vi "UHR-Fleezers Control (host) - 12.6.1.vi"() -> ()   [LabVIEW 2012] (continued)
                                n1136 = And(x=w1687, y=w1688) -> (x .and. y?=w1685:bool)
                                n1137 = And(x=w1686, y=w1688) -> (x .and. y?=w1684:bool)
                                n1138 = case shown="True" w1685 {
                                frame False {
                                }
                                frame True {
                                n1139 = local read "Confocal Y 2 (V)"() -> (w1694:dbl)
                                n1140 = local read "Confocal X 2 (V)"() -> (w1693:dbl)
                                n1141 = property on="AO2" class="Slide (strict)"("Val(Sgnl)"=w1693) -> ()  [unwired: 2 in, 2 out]
                                n1142 = property on="AO1" class="Slide (strict)"("Val(Sgnl)"=w1694) -> ()  [unwired: 2 in, 2 out]
                                }
                                }
                                n1143 = case shown="True" w1684 {
                                frame False {
                                }
                                frame True {
                                n1144 = local read "Confocal X 1 (V)"() -> (w1691:dbl)
                                n1145 = local read "Confocal Y 1 (V)"() -> (w1692:dbl)
                                n1146 = property on="AO1" class="Slide (strict)"("Val(Sgnl)"=w1692) -> ()  [unwired: 2 in, 2 out]
                                n1147 = property on="AO2" class="Slide (strict)"("Val(Sgnl)"=w1691) -> ()  [unwired: 2 in, 2 out]
                                }
                                }
                                }
                                frame #5 {
                                n1148 = Wait (ms)(milliseconds to wait=u32 1500) -> ()  [unwired: 1 out]
                                }
                                frame #6 {
                                n1149 = property on="Rem fb disp offset" class="Bool (strict)"("Val(Sgnl)"=TRUE ("Value (Signaling)")) -> ()  [unwired: 2 in, 2 out]
                                }
                                }
                                }
                                frame True {
                                n1150 = flat-sequence {
                                tunnel: w1697 -> [w1698]
                                frame #0 {
                                n1151 = property on="Trap Delta (MHz)" class="DigNum (strict)"("Val(Sgnl)"=w1698) -> ()  [unwired: 2 in, 2 out]
                                }
                                frame #1 {
                                n1152 = Wait (ms)(milliseconds to wait=u32 500) -> ()  [unwired: 1 out]
                                }
                                frame #2 {
                                n1153 = local read "Shift confocal"() -> (w1704:bool)
                                n1154 = local read "Mean"() -> (w1706:dbl)
                                n1155 = Greater?(x=w1706, y=11.0) -> (0:w1703:bool)
                                n1156 = Not(x=w1703) -> (.not. x?=w1702:bool)
                                n1157 = And(x=w1703, y=w1704) -> (x .and. y?=w1701:bool)
                                n1158 = And(x=w1702, y=w1704) -> (x .and. y?=w1700:bool)
                                n1159 = case shown="True" w1701 {
                                frame False {
                                }
                                frame True {
                                n1160 = local read "Confocal Y 2 (V)"() -> (w1710:dbl)
                                n1161 = local read "Confocal X 2 (V)"() -> (w1709:dbl)
                                n1162 = property on="AO2" class="Slide (strict)"("Val(Sgnl)"=w1709) -> ()  [unwired: 2 in, 2 out]
                                n1163 = property on="AO1" class="Slide (strict)"("Val(Sgnl)"=w1710) -> ()  [unwired: 2 in, 2 out]
                                }
                                }
                                n1164 = case shown="True" w1700 {
                                frame False {
                                }
                                frame True {
                                n1165 = local read "Confocal Y 1 (V)"() -> (w1708:dbl)
                                n1166 = local read "Confocal X 1 (V)"() -> (w1707:dbl)
                                n1167 = property on="AO2" class="Slide (strict)"("Val(Sgnl)"=w1707) -> ()  [unwired: 2 in, 2 out]
                                n1168 = property on="AO1" class="Slide (strict)"("Val(Sgnl)"=w1708) -> ()  [unwired: 2 in, 2 out]
                                }
                                }
                                }
                                }
                                }
                                }
                                }
                                }
                                }
                                }
                                n1169 = local read "Messages"() -> (w1656:string)
                                n1170 = Subtract(x=w1648, y=w1647) -> (x-y=w1654:dbl)
                                "Duration (s)" <- w1654
                                n1171 = Number To Decimal String(number=w1654, width (-)=i16 0) -> (decimal integer string=w1652:string)
                                n1172 = Concatenate Strings(w1652, " s fluorescence event." ("string")) -> (w1650:string)
                                n1173 = call "Update messages.vi"("Message to add"=w1650, "Old message string"=w1656) -> ("New message string"=w1655:string)
                                n1174 = local write "Reset Force"(FALSE ("Reset Force")) -> ()
                                n1175 = local write "Waiting"(TRUE ("Waiting")) -> ()
                                n1176 = local write "Messages"(w1655) -> ()
                                n1177 = local write "Fl. High"(FALSE ("Fl. High")) -> ()
                                n1178 = call <vilib>:"Beep.vi"() -> ()  [unwired: 3 in, 9 out]
                                }
                                }
                                n1179 = node-c288() -> ()  [unwired: 2 out]
                              }
                              n1180 = node-c288(w1624) -> ()  [unwired: 1 out]
                            }
                          }
                        }
                      }
                      n1181 = local read "Trap Delta (MHz)"() -> (w1539:dbl)
                      n1182 = local read "Trap Pos FB SP"() -> (w1534:fxp<+/-,16,1>)
                    }
                  }
                }
                frame #1 {
                  n1183 = local read "Stop All"() -> (w1720:bool)
                  n1184 = local read "Fl. Triggered..."() -> (w1718:bool)
                  n1185 = Not(x=w1718) -> (.not. x?=w1719:bool)
                  n1186 = Or(x=w1719, y=w1720) -> (x .or. y?=w1717:bool)
                }
              }
              n1187 = case shown="True" w1311 {
                frame False {
                }
                frame True {
                  n1188 = local read "Confocal Y 1 (V)"() -> (w1321:dbl)
                  n1189 = local read "Confocal X 1 (V)"() -> (w1320:dbl)
                  n1190 = property on="AO2" class="Slide (strict)"("Val(Sgnl)"=w1320) -> ()  [unwired: 2 in, 2 out]
                  n1191 = property on="AO1" class="Slide (strict)"("Val(Sgnl)"=w1321) -> ()  [unwired: 2 in, 2 out]
                }
              }
              n1192 = case shown="True" w1311 {
                frame False {
                }
                frame True {
                  w1319 = FALSE ("Fl. High")
                  n1193 = local write "Waiting"(w1319) -> ()
                  n1194 = local write "Fl. High"(w1319) -> ()
                }
              }
              n1195 = node-c288() -> ()  [unwired: 2 out]
            }
            n1196 = node-c288(w1309) -> ()  [unwired: 1 out]
          }
        }
      }
      event "Stop All": Value Change {
        n1197 = event-data() -> ()  [unwired: 7 out]
        n1198 = local read "Stop All"() -> (w1725:bool)
      }
    }
    n1199 = node-c288() -> ()  [unwired: 2 out]
  }
  n1200 = timed-loop "Basic control parameters (all FPGA settings, other basic controls)" {
    tunnel: w17 -> [w1734]
    shift-right: [w1733] -> _
    shift-left: errorcluster {"status"=FALSE, "code"=0, "source"=""} ("error out") -> [w1732]
    tunnel: [w1731] -> _
    timing: w127 -> [_]
    timing-out: [_] -> w126
    tunnel: w100 -> [w1730]
    tunnel: w72 -> [w1729]
    tunnel: w71 -> [w1728]
    tunnel: w70 -> [w1727]
    tunnel: w69 -> [w1726]
    stop <- w1731 stop-if-true
    n1201 = node-c288() -> ()  [unwired: 2 out]
    n1202 = event shown="[4] \"- phase (DIO)\", \"+ phase (AI1)\", \"- phase (AI1)\", \"Phase adj. (DIO)\", \"+ phase (DIO)\": Value Change" {
      selector: _ -> [_ _ _ _ _ _ _ _ _ _ _ _ _ _ _ _ _ _ _ _ _ _ _ _ _ _ _ _ _ _ _ _ _ _ _ _ _ _ _ _ _ _ _ _ _ _ _ _ _ _ _ _ _ _ _ _ _ _ _ _ _ _ _ _ _ _ _ _ _ _ _ _ _ _]
      dyn-events: _ -> [_ _ _ _ _ _ _ _ _ _ _ _ _ _ _ _ _ _ _ _ _ _ _ _ _ _ _ _ _ _ _ _ _ _ _ _ _ _ _ _ _ _ _ _ _ _ _ _ _ _ _ _ _ _ _ _ _ _ _ _ _ _ _ _ _ _ _ _ _ _ _ _ _ _]
      timeout: _ -> [_ _ _ _ _ _ _ _ _ _ _ _ _ _ _ _ _ _ _ _ _ _ _ _ _ _ _ _ _ _ _ _ _ _ _ _ _ _ _ _ _ _ _ _ _ _ _ _ _ _ _ _ _ _ _ _ _ _ _ _ _ _ _ _ _ _ _ _ _ _ _ _ _ _]
      tunnel: w1734 -> [w1775 _ _ _ w1819 _ w1841 _ _ _ _ w1907 _ _ w1950 w1956 w1963 w1968 w2041 _ w2057 w2082 w2103 w2124 w2144 w2173 w2199 w2202 w2206 w2301 w2306 w2344 _ w2379 w2383 w2394 w2398 w2402 _ w2410 _ _ _ _ _ _ _ _ _ _ _ _ _ _ _ _ _ w2788 _ w2805 _ w2812 w2830 _ w2837 w2845 w2860 w2876 w2882 _ w2891 _ w2910 _]
      tunnel: [w1774 _ _ _ w1809 _ w1840 _ _ w1872 _ w1886 _ _ w1949 w1952 w1962 w1965 w2035 _ w2056 w2081 w2101 w2122 w2142 w2167 w2197 _ w2204 w2299 w2304 w2342 _ w2377 w2381 w2385 w2396 w2400 _ w2408 _ _ _ _ _ _ _ _ _ _ _ _ _ _ _ _ _ w2786 _ _ _ _ w2827 _ _ _ _ _ _ _ _ _ _ _] -> w1733
      tunnel: w1732 -> [w1773 _ _ _ w1818 _ w1839 _ _ w1872 _ w1906 _ _ w1948 w1951 w1961 w1964 w2040 _ w2055 w2080 w2102 w2123 w2143 w2172 w2198 w2201 w2205 w2300 w2305 w2343 _ w2378 w2382 w2393 w2397 w2401 _ w2409 _ _ _ _ _ _ _ _ _ _ _ _ _ _ _ _ _ w2787 _ w2804 _ w2811 w2829 _ w2836 w2844 w2859 w2875 w2881 _ w2890 _ w2909 _]
      tunnel: [_ _ _ _ _ _ _ _ _ w1871 _ _ _ _ _ _ _ _ _ _ _ _ _ _ _ _ _ _ _ _ _ _ _ _ _ _ _ _ _ _ _ _ _ _ _ _ _ _ _ _ _ _ _ _ _ _ _ _ _ _ _ _ _ _ _ _ _ _ _ _ _ _ _ _] -> w1731
      tunnel: [_ _ _ _ _ _ _ "Round T1 X" _ _ _ _ _ _ _ _ _ _ _ _ _ _ _ _ _ _ _ _ _ _ _ _ _ _ _ _ _ _ _ _ _ _ _ _ _ _ _ _ _ _ _ _ _ _ _ _ _ _ _ _ _ _ _ _ _ _ _ _ _ _ _ _ _ _] -> _
      tunnel: [_ _ _ "Adjust Scale\nto Mean" _ _ _ _ _ _ _ _ _ _ _ _ _ _ _ _ _ _ _ _ _ _ _ _ "Test ttrig" _ _ _ _ _ _ _ _ _ _ _ _ _ _ _ _ _ _ "Flush Sample" "Flush Pump 3" "Flush Pump 1" "Clear Volume" _ _ _ _ _ _ _ _ _ _ _ _ _ _ _ _ _ _ _ _ _ _ _] -> _
      tunnel: [_ _ _ _ _ _ _ _ "Round T2 X" _ "Delayed Interlace Start" _ _ _ _ _ _ _ _ _ _ _ _ _ _ _ _ _ _ _ _ _ _ _ _ _ _ _ _ _ _ _ _ _ _ _ _ _ _ _ _ _ _ _ _ _ _ _ _ _ _ _ _ _ _ _ _ _ _ _ _ _ _ _] -> _
      tunnel: w1730 -> [_ _ _ _ _ _ _ _ _ _ _ _ _ _ _ _ _ _ _ _ _ _ _ _ _ _ _ _ _ _ _ _ _ _ _ _ _ _ _ _ _ _ _ w2567 w2574 w2581 w2586 w2595 _ _ w2701 _ _ _ _ _ _ _ _ _ _ _ _ _ _ _ _ _ _ _ _ _ _ _]
      tunnel: w1729 -> [_ _ _ _ _ _ _ _ _ _ _ _ _ _ _ _ _ _ _ _ _ _ _ _ _ _ _ _ _ _ _ _ _ _ _ _ _ _ _ _ _ w2484 _ _ _ _ _ _ w2639 _ _ w2707 _ w2716 _ w2730 _ _ _ _ _ _ _ _ _ _ _ _ _ _ _ _ _ _]
      tunnel: w1728 -> [_ _ _ _ _ _ _ _ _ _ _ _ _ _ _ _ _ _ _ _ _ _ _ _ _ _ _ _ _ _ _ _ _ _ _ _ _ _ _ _ _ _ _ _ _ _ _ _ _ _ _ _ _ _ _ _ _ _ _ _ _ _ _ _ _ _ _ _ _ _ _ _ _ _]
      tunnel: w1727 -> [_ _ _ _ _ _ _ _ _ _ _ _ _ _ _ _ _ _ _ _ _ _ _ _ _ _ _ _ _ _ _ _ _ _ _ _ _ _ _ _ w2421 _ _ _ _ _ _ _ _ w2669 _ _ w2712 _ w2723 _ w2755 _ _ _ _ _ _ _ _ _ _ _ _ _ _ _ _ _]
      tunnel: w1726 -> [_ _ _ _ _ _ _ _ _ _ _ _ _ _ _ _ _ _ _ _ _ _ _ _ _ _ _ _ _ _ _ _ _ _ _ _ _ _ _ _ _ _ _ _ _ _ _ _ _ _ _ _ _ _ _ _ _ _ _ _ _ _ _ _ _ _ _ _ _ _ _ _ _ _]
      event "AI Count (ticks)", "Sets to FIFO (Traps)", "Save ave N", "FPGA Ave.", "# Samples/channel", "N sets to save": Value Change {
        # "So that if 'Save ave N' is updated, the AOD scanning code updates too."
        n1203 = event-data() -> ()  [unwired: 6 out]
        n1204 = local read "AI Count (ticks)"() -> (w1757:u16)
        n1205 = Unbundle By Name("Sets to FIFO (Traps)") -> ("Set 1"=w1740:bool, "Set 2"=w1739:bool, "Set 3"=w1738:bool)
        n1206 = Boolean To (0,1)(Boolean="Sets to FIFO (Traps)") -> (0, 1=w1765:cluster{"Set 1":i16, "Set 2":i16, "Set 3":i16})
        n1207 = xnode "Read/Write Control"("FPGA VI Reference In"=w1775, "error in"=w1773, "ai count"=w1757, "Set 1"=w1740, "Set 2"=w1739, "Set 3"=w1738, "N of AI1 Int Acq Sets"="N Acq Sets (Traps + Fl.)") -> ("error out"=w1774:errorcluster)  [unwired: 1 out]
        n1208 = Cluster To Array(cluster=w1765) -> (array=w1764:i16[])
        n1209 = To Unsigned Long Integer(number=w1764) -> (unsigned 32bit integer=w1746:u32[])
        n1210 = local read "Scan steps (AOD)"() -> (w1766:u64)
        n1211 = Multiply(x=w1757, y="N Acq Sets (Traps + Fl.)") -> (x*y=w1755:u16)
        n1212 = Divide(x=40000000.0, y=w1757) -> (x/y=w1749:dbl)
        "AI rate (Hz)" <- w1749
        "Ave. Rate (Hz)" <- w1749
        n1213 = Add Array Elements(numeric array=w1746) -> (sum=w1758:u32)
        "Trap Sets" <- w1758
        n1214 = Reciprocal(x=w1749) -> (1/x=→"Ave. Period (s)":dbl)
        n1215 = property on="Scan steps (AOD)" class="DigNum (strict)"("Val(Sgnl)"=w1766) -> ()  [unwired: 2 in, 2 out]
        n1216 = Divide(x=w1749, y="N Acq Sets (Traps + Fl.)") -> (x/y=w1770:dbl)
        "Data Rate (Hz)" <- w1770
        n1217 = Reciprocal(x=w1770) -> (1/x=→"Data Period (s)":dbl)
        n1218 = local read "Save ave N"() -> (w1769:dbl)
        n1219 = Divide(x=w1770, y=w1769) -> (x/y=w1768:dbl)
        "Save Data Rate (Hz)" <- w1768
        n1220 = Reciprocal(x=w1768) -> (1/x=→"Save Data Period (s)":dbl)
        n1221 = Multiply(x=w1755, y="# Samples/trap") -> (x*y=w1753:u32)
        "Counts/DMA" <- w1753
        n1222 = property on="Trap Disp. Downsample" class="DigNum (strict)"("Maximum"="# Samples/trap") -> ()  [unwired: 2 in, 2 out]
        n1223 = Multiply(x=w1758, y="# Samples/trap") -> (x*y=w1747:u32)
        "# Samples/channel" <- w1747
        n1224 = Multiply(x=w1747, y=u32 8) -> (x*y=→"Trap AI Elements/DMA read":u32)
        n1225 = local read "APD Int. Count"() -> (w1754:u32)
        n1226 = Multiply(x=w1747, y=u32 3) -> (x*y=→"Trap Pos Elements/DMA read":u32)
        n1227 = Divide(x=w1753, y=w1754) -> (x/y=w1744:dbl)
        "APD Samples/FIFO Acq." <- w1744
        n1228 = Divide(x=w1753, y=40000000.0) -> (x/y=w1751:dbl)
        "DMA Update Period (s)" <- w1751
        n1229 = local read "Number of APDs"() -> (w1737:u8)
        n1230 = Multiply(x=w1737, y=w1744) -> (x*y=→"APD Elements/DMA read":dbl)
        n1231 = property on="APD Disp. Downsample" class="DigNum (strict)"("Maximum"=w1744) -> ()  [unwired: 2 in, 2 out]
        n1232 = local read "N sets to save"() -> (w1763:u32)
        n1233 = Multiply(x=w1751, y=w1763) -> (x*y=→"Total Time (s)":dbl)
        "FPGA Averaging" <- FALSE ("FPGA Averaging")
      }
      event "Remove Offset": Value Change {
        n1234 = event-data() -> ()  [unwired: 7 out]
        n1235 = local write "Remove Offset"(FALSE ("Remove Offset")) -> ()
        n1236 = local read "Bead Mean (nm)"() -> (w1777:dbl)
        n1237 = local read "Offset (nm)"() -> (w1778:dbl)
        n1238 = Add(x=w1777, y=w1778) -> (x+y=w1776:dbl)
        n1239 = local write "Offset (nm)"(w1776) -> ()
        n1240 = disable-structure shown="Disabled" {
          frame Disabled {
            n1241 = local read "Bead Mean (nm)"() -> (w1783:dbl)
            n1242 = Add(y=w1783) -> (x=w1782:dbl, x+y=w1781:dbl)
            n1243 = Subtract(x=w1783, y=w1782) -> (x-y=w1780:dbl)
            n1244 = property on="Bead Separation" class="WFChart (strict)"("YScale.Minimum"=w1780) -> ()  [unwired: 2 in, 2 out]
            n1245 = property on="Bead Separation" class="WFChart (strict)"("YScale.Maximum"=w1781) -> ()  [unwired: 2 in, 2 out]
          }
          frame Enabled {
          }
        }
      }
      event "Detector Type": Value Change {
        n1246 = event-data() -> ()  [unwired: 7 out]
        n1247 = local read "AI labels"() -> (w1784:string[])
        n1248 = property on="High Res. Display" class="Ring (strict)"("Strings []"=w1784) -> ()  [unwired: 2 in, 2 out]
        n1249 = Build Array (concatenate)(w1784, "none") -> (w1785:string[])
        n1250 = property on="FFT 1 Choice 1" class="Ring (strict)"("Strings []"=w1785) -> ()  [unwired: 2 in, 2 out]
        n1251 = property on="FFT 1 Choice 2" class="Ring (strict)"("Strings []"=w1785) -> ()  [unwired: 2 in, 2 out]
        n1252 = property on="FFT 2 Choice 1" class="Ring (strict)"("Strings []"=w1785) -> ()  [unwired: 2 in, 2 out]
        n1253 = property on="FFT 2 Choice 2" class="Ring (strict)"("Strings []"=w1785) -> ()  [unwired: 2 in, 2 out]
        n1254 = Bundle("APD 1", "APD 2") -> (w1788:cluster{string, string})  [unwired: 1 out]
        n1255 = Cluster To Array(cluster=w1788) -> (array=w1786:string[])
        n1256 = Build Array (concatenate)(w1786, w1785) -> (w1790:string[])
        n1257 = Array Size(array=w1790) -> (size(s)=w1791:i32)
        n1258 = property on="Signals to Plot" class="LstBox (strict)"("Item Names"=w1790) -> ()  [unwired: 2 in, 2 out]
        n1259 = property on="Signals to Plot" class="LstBox (strict)"("Number of Rows"=w1791) -> ()  [unwired: 2 in, 2 out]
        n1260 = property on="All Signals" class="WFChart (strict)"("LegNumRows"=w1791) -> ()  [unwired: 2 in, 2 out]
      }
      event "Adjust Scale\nto Mean": Value Change {
        n1261 = event-data() -> ()  [unwired: 7 out]
        n1262 = local read "APD 1 Rate (Hz)"() -> (w1800:dbl)
        n1263 = Multiply(x=1000.0, y="Above (kHz)") -> (x*y=w1798:dbl)
        n1264 = Multiply(x=1000.0, y="Below (kHz)") -> (x*y=w1796:dbl)
        n1265 = Add(x=w1798, y=w1800) -> (x+y=w1793:dbl)
        n1266 = Subtract(x=w1800, y=w1796) -> (x-y=w1794:dbl)
        n1267 = property on="APD Chart" class="WFChart (strict)"("YScale.Minimum"=w1794) -> ()  [unwired: 2 in, 2 out]
        n1268 = property on="APD Chart" class="WFChart (strict)"("YScale.Maximum"=w1793) -> ()  [unwired: 2 in, 2 out]
      }
      event "- phase (DIO)", "+ phase (AI1)", "- phase (AI1)", "Phase adj. (DIO)", "+ phase (DIO)": Value Change {
        # "digital phase (controls switching phase of AOM/AOD)"
        # "Analog phase"
        n1269 = event-data() -> ()  [unwired: 7 out]
        n1270 = Negate(x="Phase adj. (AI1)") -> (-x=w1816:i16)
        n1271 = Negate(x="Phase adj. (DIO)") -> (-x=w1805:i16)
        n1272 = Select(t=w1816, s="- phase (AI1)", f="Phase adj. (AI1)") -> (s? t:f=w1815:i16)
        n1273 = Select(t=w1805, s="- phase (DIO)", f="Phase adj. (DIO)") -> (s? t:f=w1804:i16)
        n1274 = xnode "Read/Write Control"("FPGA VI Reference In"=w1819, "error in"=w1818, "Phase count adjustment"=w1815, "Phase count adjustment (DIO)"=w1804) -> ("FPGA VI Reference Out"=w1814:T20, "error out"=w1813:errorcluster)
        n1275 = Or(x="- phase (AI1)", y="+ phase (AI1)") -> (x .or. y?=w1810:bool)
        n1276 = Or(x="- phase (DIO)", y="+ phase (DIO)") -> (x .or. y?=w1808:bool)
        n1277 = xnode "Read/Write Control"("FPGA VI Reference In"=w1814, "error in"=w1813, "+ phase"=w1810, "+ phase (DIO)"=w1808) -> ("error out"=w1809:errorcluster)  [unwired: 1 out]
      }
      event "Signals to Plot": Double Click {
        w1822 = u32 9868950 ("Color Box")
        n1278 = event-data() -> ("Row"=w1824:i32)  [unwired: 9 out]
        n1279 = property on="All Signals" class="WFChart (strict)"("Active Plot"=w1824) -> (error out=w1835:errorcluster)  [unwired: 2 in, 1 out]
        n1280 = property on="All Signals" class="WFChart (strict)" props=["Plot", "Visible?", "Plot", "Plot Color"](error in=w1835) -> (error out=w1834:errorcluster, "Plot.Visible?"=w1833:bool)  [unwired: 1 in, 2 out]
        n1281 = Select(t=FALSE ("Plot.Visible"), s=w1833, f=TRUE ("Plot.Visible")) -> (s? t:f=w1828:bool)
        n1282 = property on="All Signals" class="WFChart (strict)"(error in=w1834, "Plot.Visible?"=w1828) -> (error out=w1830:errorcluster)  [unwired: 1 in, 1 out]
        n1283 = property on="All Signals" class="WFChart (strict)"(error in=w1830) -> (error out=w1825:errorcluster, "Plot.Plot Color"=w1829:u32)  [unwired: 1 in, 1 out]
        n1284 = property on="Signals to Plot" class="LstBox (strict)"(error in=w1825, "Active Row"=w1824) -> (error out=w1823:errorcluster)  [unwired: 1 in, 1 out]
        n1285 = Select(t=w1829, s=w1828, f=u32 0) -> (s? t:f=w1826:u32)
        n1286 = property on="Signals to Plot" class="LstBox (strict)"(error in=w1823, "CellFontColor"=w1826, "SelColor"=w1822, "CellBG"=w1822, "CellFontSize"=u32 20 ("Active Row:Cell Font:Size"), "CellFontBold"=TRUE ("Active Row:Cell Font:Bold")) -> ()  [unwired: 1 in, 2 out]
      }
      event "BD 1 Frequency 1 (MHz)", "BD 1 Frequency 2 (MHz)", "BD 1 Frequency 3 (MHz)", "BD 2 Frequency 1 (MHz)", "BD 2 Frequency 2 (MHz)", "BD 2 Frequency 3 (MHz)", "Trap Delta (MHz)": Value Change {
        n1287 = event-data() -> ("CtlRef"=w1838:refnum<vi>)  [unwired: 6 out]
        n1288 = control-ref of="Trap Delta (MHz)"() -> (w1837:refnum<vi>)
        n1289 = Equal?(x=w1837, y=w1838) -> (x = y?=w1836:bool)
        n1290 = case shown="False" "Oscillate Set 1" {
          tunnel: w1841 -> [w1861 _]
          tunnel: [w1860 w1864] -> w1840
          tunnel: w1839 -> [w1859 w1864]
          tunnel: w1836 -> [w1844 _]
          frame False {
            n1291 = local read "BD 1 Frequency 2 (MHz)"() -> (w1848:dbl)
            n1292 = local read "BD 1 Frequency 1 (MHz)"() -> (w1846:dbl)
            n1293 = Subtract(x=w1848, y="Trap Delta (MHz)") -> (x-y=w1845:dbl)
            n1294 = Select(t=w1845, s=w1844, f=w1846) -> (s? t:f=w1843:dbl)
            n1295 = local read "Y RF Frequency Limits (MHz)"() -> (w1849:T16)
            n1296 = local read "X RF Frequency Limits (MHz)"() -> (w1850:T16)
            n1297 = local read "BD 1 Frequency 3 (MHz)"() -> (w1862:dbl)
            n1298 = local write "BD 1 Frequency 1 (MHz)"(w1843) -> ()
            n1299 = local read "BD 2 Frequency 1 (MHz)"() -> (w1853:dbl)
            n1300 = local read "BD 2 Frequency 2 (MHz)"() -> (w1852:dbl)
            n1301 = local read "BD 2 Frequency 3 (MHz)"() -> (w1863:dbl)
            n1302 = call "set RF board frequency - interlace.vi"("Board 2 Frequency Limits"=w1849, "Board 1 Frequency Limits"=w1850, "error in"=w1859, "FPGA VI Reference In"=w1861, "Board 2 Frequency 3 (MHz)"=w1863, "Board 1 Frequency 3 (MHz)"=w1862, "Board 2 Frequency 2 (MHz)"=w1852, "Board 2 Frequency 1 (MHz)"=w1853, "Board 1 Frequency 2 (MHz)"=w1848, "Board 1 Frequency 1  (MHz)"=w1843) -> ("error out"=w1860:errorcluster)  [unwired: 1 out]
            n1303 = Subtract(x=w1853, y=w1852) -> (x-y=w1857:dbl)
            n1304 = Subtract(x=w1843, y=w1848) -> (x-y=w1858:dbl)
            n1305 = Square(x=w1857) -> (x^2=w1855:dbl)
            n1306 = Square(x=w1858) -> (x^2=w1856:dbl)
            n1307 = Add(x=w1856, y=w1855) -> (x+y=w1854:dbl)
            n1308 = Square Root(x=w1854) -> (sqrt(x)=w1851:dbl)
            n1309 = local write "Trap Delta (MHz)"(w1851) -> ()
            n1310 = property on="Initial delta (MHz)" class="DigNum (strict)"("Val(Sgnl)"=w1851) -> ()  [unwired: 2 in, 2 out]
          }
          frame True {
          }
        }
      }
      event "Round T1 X": Value Change {
        n1311 = event-data() -> ()  [unwired: 7 out]
        n1312 = local read "BD 1 Frequency 1 (MHz)"() -> (w1867:dbl)
        n1313 = Round To Nearest(number=w1867) -> (nearest integer value=w1866:dbl)
        n1314 = property on="BD 1 Frequency 1 (MHz)" class="DigNum (strict)"("Val(Sgnl)"=w1866) -> ()  [unwired: 2 in, 2 out]
      }
      event "Round T2 X": Value Change {
        n1315 = event-data() -> ()  [unwired: 7 out]
        n1316 = local read "BD 1 Frequency 2 (MHz)"() -> (w1869:dbl)
        n1317 = Round To Nearest(number=w1869) -> (nearest integer value=w1868:dbl)
        n1318 = property on="BD 1 Frequency 2 (MHz)" class="DigNum (strict)"("Val(Sgnl)"=w1868) -> ()  [unwired: 2 in, 2 out]
      }
      event "Stop All": Value Change {
        n1319 = event-data() -> ()  [unwired: 7 out]
        n1320 = local read "Stop All"() -> (w1871:bool)
      }
      event "Delayed Interlace Start": Value Change {
        n1321 = event-data() -> ()  [unwired: 7 out]
        n1322 = flat-sequence {
          frame #0 {
            n1323 = Multiply(x="Delay to Interlace (s)", y=1000.0) -> (x*y=w1874:dbl)
            n1324 = Wait (ms)(milliseconds to wait=w1874) -> ()  [unwired: 1 out]
          }
          frame #1 {
            n1325 = property on="Laser interlacing mode" class="RadioBtnsControl (strict)"("Val(Sgnl)"=enum32{"Laser ON", "Laser OFF", "Interlace"}."Interlace" ("Value (Signaling)")) -> ()  [unwired: 2 in, 2 out]
          }
        }
      }
      event "BD 1 Amplitude 1 (%)", "BD 1 Amplitude 2 (%)", "BD 1 Amplitude 3 (%)", "BD 2 Amplitude 1 (%)", "BD 2 Amplitude 2 (%)", "BD 2 Amplitude 3 (%)", "Trap 1 ON", "Trap 2 ON", "Trap 3 ON", "Feedback On/Off", "All FB On/Off": Value Change {
        w1898 = i16 1 ("f")
        n1326 = event-data() -> ()  [unwired: 7 out]
        n1327 = local write "Trap 1 (ON/OFF)"("Trap 1 ON") -> ()
        n1328 = local write "Trap 2 (ON/OFF)"("Trap 2 ON") -> ()
        n1329 = Boolean To (0,1)(Boolean="Trap 3 ON") -> (0, 1=w1899:i16)
        n1330 = Boolean To (0,1)(Boolean="Trap 1 ON") -> (0, 1=w1900:i16)
        n1331 = Boolean To (0,1)(Boolean="Trap 2 ON") -> (0, 1=w1901:i16)
        n1332 = Select(t=w1901, s="Trap ON/OFF X or Y Amp?", f=w1898) -> (s? t:f=w1896:i16)
        n1333 = Select(t=w1900, s="Trap ON/OFF X or Y Amp?", f=w1898) -> (s? t:f=w1897:i16)
        n1334 = Select(t=w1899, s="Trap ON/OFF X or Y Amp?", f=w1898) -> (s? t:f=w1895:i16)
        n1335 = Select(t=w1898, s="Trap ON/OFF X or Y Amp?", f=w1901) -> (s? t:f=w1893:i16)
        n1336 = Select(t=w1898, s="Trap ON/OFF X or Y Amp?", f=w1900) -> (s? t:f=w1894:i16)
        n1337 = Select(t=w1898, s="Trap ON/OFF X or Y Amp?", f=w1899) -> (s? t:f=w1892:i16)
        n1338 = And(x="All FB On/Off", y="Feedback On/Off") -> (x .and. y?=w1890:cluster{"Set 1":bool, "Set 2":bool})
        n1339 = local read "BD 1 Amplitude 1 (%)"() -> (w1910:dbl)
        n1340 = local read "BD 1 Amplitude 2 (%)"() -> (w1909:dbl)
        n1341 = local read "BD 1 Amplitude 3 (%)"() -> (w1908:dbl)
        n1342 = Unbundle By Name(w1890) -> ("Set 1"=w1885:bool, "Set 2"=w1882:bool)
        n1343 = local read "Y RF Amplitude Limits (%)"() -> (w1878:T16)
        n1344 = local read "X RF Amplitude Limits (%)"() -> (w1879:T16)
        n1345 = local read "BD 2 Amplitude 1 (%)"() -> (w1911:dbl)
        n1346 = local read "BD 2 Amplitude 2 (%)"() -> (w1912:dbl)
        n1347 = local read "BD 2 Amplitude 3 (%)"() -> (w1913:dbl)
        n1348 = And(x="Trap 2 ON", y=w1882) -> (x .and. y?=w1880:bool)
        n1349 = And(x="Trap 1 ON", y=w1885) -> (x .and. y?=w1883:bool)
        n1350 = Multiply(x=w1897, y=w1910) -> (x*y=w1905:dbl)
        n1351 = Multiply(x=w1909, y=w1896) -> (x*y=w1903:dbl)
        n1352 = Multiply(x=w1908, y=w1895) -> (x*y=w1904:dbl)
        n1353 = Multiply(x=w1911, y=w1894) -> (x*y=w1914:dbl)
        n1354 = Multiply(x=w1912, y=w1893) -> (x*y=w1915:dbl)
        n1355 = Multiply(x=w1913, y=w1892) -> (x*y=w1916:dbl)
        n1356 = call "set RF board amplitude - interlace.vi"("Board 2 Amplitude Limits"=w1878, "Board 1 Amplitude Limits"=w1879, "error in"=w1906, "FPGA VI Reference In"=w1907, "Board 2 Amplitude 3 (%)"=w1916, "Board 1 Amplitude 3 (%)"=w1904, "Board 2 Amplitude 2 (%)"=w1915, "Board 2 Amplitude 1 (%)"=w1914, "Board 1 Amplitude 2 (%)"=w1903, "Board 1 Amplitude 1 (%)"=w1905) -> ("error out"=w1887:errorcluster, "FPGA VI Reference Out"=w1888:T20)
        n1357 = xnode "Read/Write Control"("FPGA VI Reference In"=w1888, "error in"=w1887, "FB On/Off Set 1"=w1883, "FB On/Off Set 2"=w1880) -> ("error out"=w1886:errorcluster)  [unwired: 1 out]
      }
      event "Load parameters": Value Change {
        n1358 = event-data() -> ()  [unwired: 7 out]
        n1359 = property on="Saved AOD Raster Scan Parameter Sets" class="Arr (strict)"() -> ("Index Values"=w1927:u32[])  [unwired: 2 in, 2 out]
        n1360 = Index Array(array=w1927, index=0) -> (element=w1924:u32)
        n1361 = local write "Load parameters"(FALSE ("Load parameters")) -> ()
        n1362 = Index Array(array="Saved AOD Raster Scan Parameter Sets", index=w1924) -> (element=w1923:T30)
        n1363 = Unbundle By Name(w1923) -> ("Scan Range AOD (nm) 2"=w1922:dbl, "Step Size AOD (nm) 2"=w1921:dbl, "Scan Speed AOD (nm/s) 2"=w1920:dbl, "Number of scans (AOD) 2"=w1919:u16)
        n1364 = flat-sequence {
          tunnel: w1922 -> [w1930]
          tunnel: w1921 -> [w1929]
          tunnel: w1920 -> [w1928]
          tunnel: w1919 -> [w1931]
          frame #0 {
            n1365 = local write "Scan Speed (nm/s)"(w1928) -> ()
            n1366 = local write "Scan Range (nm)"(w1930) -> ()
            n1367 = local write "Step Size (nm)"(w1929) -> ()
          }
          frame #1 {
            n1368 = property on="Number of F/B Scans (AOD)" class="DigNum (strict)"("Val(Sgnl)"=w1931) -> ()  [unwired: 2 in, 2 out]
          }
        }
      }
      event "Trap 1 (ON/OFF)", "Trap 2 (ON/OFF)": Value Change {
        n1369 = event-data() -> ()  [unwired: 7 out]
        n1370 = property on="Trap 2 ON" class="Bool (strict)"("Val(Sgnl)"="Trap 2 (ON/OFF)") -> ()  [unwired: 2 in, 2 out]
        n1371 = property on="Trap 1 ON" class="Bool (strict)"("Val(Sgnl)"="Trap 1 (ON/OFF)") -> ()  [unwired: 2 in, 2 out]
      }
      event "DIO count 1 (ticks)", "DIO count 2 (ticks)", "DIO count 3 (ticks)", "Interlace", "Number Interlace Sets", "Not-Interlacing Set": Value Change {
        n1372 = event-data() -> ()  [unwired: 7 out]
        n1373 = local read "DIO count 3 (ticks)"() -> (w1944:u16)
        n1374 = local read "DIO count 1 (ticks)"() -> (w1946:u16)
        n1375 = local read "DIO count 2 (ticks)"() -> (w1945:u16)
        n1376 = To Unsigned Byte Integer(number="Not-Interlacing Set") -> (unsigned 8bit integer=w1935:u8)
        n1377 = Add(x=w1935, y=u8 1) -> (x+y=w1939:u8)
        n1378 = xnode "Read/Write Control"("FPGA VI Reference In"=w1950, "error in"=w1948, "DIO count 1 (ticks)"=w1946, "DIO count 2 (ticks)"=w1945, "DIO count 3 (ticks)"=w1944, "Interlace ON/OFF"="Interlace", "Number Interlace Cycles"="Number Interlace Sets", "Interlace Off Parameters"=w1939) -> ("error out"=w1949:errorcluster)  [unwired: 1 out]
        n1379 = Build Array(w1946, w1945, w1944) -> (w1937:u16[])
        n1380 = Split 1D Array(array=w1937, index="Number Interlace Sets") -> (first subarray=w1947:u16[])  [unwired: 1 out]
        n1381 = Index Array(array=w1937, index=w1935) -> (element=w1936:u16)
        n1382 = Add Array Elements(numeric array=w1947) -> (sum=w1941:u16)
        n1383 = Select(t=w1941, s="Interlace", f=w1936) -> (s? t:f=→"Total Counts (ticks)":u16)
      }
      event "Reset Feedback": Value Change {
        n1384 = event-data() -> ()  [unwired: 7 out]
        n1385 = Unbundle By Name("Reset Feedback") -> ("Set 1"=w1954:bool, "Set 2"=w1953:bool)
        n1386 = xnode "Read/Write Control"("FPGA VI Reference In"=w1956, "error in"=w1951, "FB Reset Set 1"=w1954, "FB Reset Set 2"=w1953) -> ("error out"=w1952:errorcluster)  [unwired: 1 out]
      }
      event "Trap Intensity PID Gains": Value Change {
        n1387 = event-data() -> ()  [unwired: 7 out]
        n1388 = Unbundle By Name("Trap Intensity PID Gains") -> ("proportional gain (Kc)"=w1959:i16, "integral gain (Kc*Ts/Ti)"=w1958:i16, "derivative gain (Kc*Td/Ts)"=w1957:i16)
        n1389 = xnode "Read/Write Control"("FPGA VI Reference In"=w1963, "error in"=w1961, "P1"=w1959, "I1"=w1958, "D1"=w1957) -> ("error out"=w1962:errorcluster)  [unwired: 1 out]
      }
      event "AI2 to Setpoint", "Setpoints (V)": Value Change {
        n1390 = event-data() -> ()  [unwired: 7 out]
        n1391 = xnode "Read/Write Control"("FPGA VI Reference In"=w1968, "error in"=w1964) -> ("FPGA VI Reference Out"=w1967:T20, "error out"=w1966:errorcluster, "AI2 Y Sum Set 1"=w1975:i16, "AI2 Y Sum Set 2"=w1974:i16)
        n1392 = Cluster To Array(cluster="AI2 to Setpoint") -> (array=w1978:bool[])
        n1393 = local read "AI2 (V)"() -> (w1976:cluster{"Set 1":dbl, "Set 2":dbl})
        n1394 = Or Array Elements(Boolean array=w1978) -> (logical OR=w1979:bool)
        n1395 = Bundle By Name(cluster=w1976, "Set 1"=w1975, "Set 2"=w1974) -> (w1973:cluster{"Set 1":dbl, "Set 2":dbl})
        n1396 = Divide(x=w1973, y=3276.7) -> (x/y=w1972:cluster{"Set 1":dbl, "Set 2":dbl})
        "AI2 (V)" <- w1972
        n1397 = case shown="True" w1979 {
          tunnel: [w1982 w1999] -> w1971
          tunnel: "AI2 to Setpoint" -> [_ w1995]
          tunnel: "Setpoints (V)" -> [w1983 w1998]
          tunnel: w1972 -> [_ w1992]
          frame False {
            n1398 = Multiply(x=3276.7, y=w1983) -> (x*y=w1984:cluster{"Set 1":dbl, "Set 2":dbl})
            n1399 = To Word Integer(number=w1984) -> (16bit integer=w1982:cluster{"Set 1":i16, "Set 2":i16})
          }
          frame True {
            n1400 = Unbundle By Name(w1992) -> ("Set 1"=w1991:dbl, "Set 2"=w1990:dbl)
            n1401 = Unbundle By Name(w1998) -> ("Set 1"=w1997:dbl, "Set 2"=w1996:dbl)
            n1402 = Unbundle By Name(w1995) -> ("Set 1"=w1994:bool, "Set 2"=w1993:bool)
            n1403 = Select(t=w1991, s=w1994, f=w1997) -> (s? t:f=w1989:dbl)
            n1404 = Select(t=w1990, s=w1993, f=w1996) -> (s? t:f=w1988:dbl)
            n1405 = Bundle By Name(cluster=w1998, "Set 1"=w1989, "Set 2"=w1988) -> (w1986:cluster{"Set 1":dbl, "Set 2":dbl})
            n1406 = local write "Setpoints (V)"(w1986) -> ()
            n1407 = Multiply(x=3276.7, y=w1986) -> (x*y=w1987:cluster{"Set 1":dbl, "Set 2":dbl})
            n1408 = To Word Integer(number=w1987) -> (16bit integer=w1999:cluster{"Set 1":i16, "Set 2":i16})
          }
        }
        n1409 = Unbundle By Name(w1971) -> ("Set 1"=w1970:i16, "Set 2"=w1969:i16)
        n1410 = xnode "Read/Write Control"("FPGA VI Reference In"=w1967, "error in"=w1966, "FB Setpoint Set 1"=w1970, "FB Setpoint Set 2"=w1969) -> ("error out"=w1965:errorcluster)  [unwired: 1 out]
      }
      event "+ phase (GI)", "- phase (GI)", "+ phase (GI) 2", "- phase (GI) 2", "+ phase (RI)", "- phase (RI)", "+ phase (Green FB)", "- phase (Green FB)": Value Change {
        n1411 = event-data() -> ()  [unwired: 7 out]
        n1412 = Or(x="+ phase (GI)", y="- phase (GI)") -> (x .or. y?=w2034:bool)
        n1413 = Negate(x="Phase adj. (GI)") -> (-x=w2039:i16)
        n1414 = Select(t=w2039, s="+ phase (GI)", f="Phase adj. (GI)") -> (s? t:f=w2038:i16)
        n1415 = Or(x="+ phase (GI) 2", y="- phase (GI) 2") -> (x .or. y?=w2025:bool)
        n1416 = Negate(x="Phase adj. (GI) 2") -> (-x=w2030:i16)
        n1417 = Select(t=w2030, s="+ phase (GI) 2", f="Phase adj. (GI) 2") -> (s? t:f=w2026:i16)
        n1418 = Negate(x="Phase adj. (RI)") -> (-x=w2024:i16)
        n1419 = Or(x="+ phase (RI)", y="- phase (RI)") -> (x .or. y?=w2020:bool)
        n1420 = Select(t=w2024, s="+ phase (RI)", f="Phase adj. (RI)") -> (s? t:f=w2019:i16)
        n1421 = Or(x="+ phase (Green FB)", y="- phase (Green FB)") -> (x .or. y?=w2013:bool)
        n1422 = Negate(x="Phase adj. (Green FB)") -> (-x=w2018:i16)
        n1423 = Select(t=w2018, s="+ phase (Green FB)", f="Phase adj. (Green FB)") -> (s? t:f=w2014:i16)
        n1424 = Negate(x="Phase adj. (BI AO)") -> (-x=w2012:i16)
        n1425 = Or(x="+ phase (BI AO)", y="- phase (BI AO)") -> (x .or. y?=w2002:bool)
        n1426 = Select(t=w2012, s="+ phase (BI AO)", f="Phase adj. (BI AO)") -> (s? t:f=w2004:i16)
        n1427 = Negate(x="Phase adj. (BI DO)") -> (-x=w2008:i16)
        n1428 = Or(x="+ phase (BI DO)", y="- phase (BI DO)") -> (x .or. y?=w2001:bool)
        n1429 = Select(t=w2008, s="+ phase (BI DO)", f="Phase adj. (BI DO)") -> (s? t:f=w2003:i16)
        n1430 = xnode "Read/Write Control"("FPGA VI Reference In"=w2041, "error in"=w2040, "Phase count adjustment (GI)"=w2038, "Phase count adjustment (GI) 2"=w2026, "Phase count adjustment (RI)"=w2019, "Phase count adjustment (Green FB)"=w2014, "Phase count adjustment (BI AO)"=w2004, "Phase count adjustment (BI D)"=w2003) -> ("FPGA VI Reference Out"=w2036:T20, "error out"=w2037:errorcluster)
        n1431 = xnode "Read/Write Control"("FPGA VI Reference In"=w2036, "error in"=w2037, "+ phase (GI)"=w2034, "+ phase (GI) 2"=w2025, "+ phase (RI)"=w2020, "+ phase (Green FB)"=w2013, "+ phase (BI AO)"=w2002, "+ phase (BI D)"=w2001) -> ("error out"=w2035:errorcluster)  [unwired: 1 out]
      }
      event "Green Laser ON/OFF", "Red Laser ON/OFF", "Blue Laser ON/OFF": Value Change {
        # "This loop shouldn't be initialized.  The main 'laser ON' settings should dominate and set the others."
        n1432 = event-data() -> ()  [unwired: 7 out]
        n1433 = property on="Red Laser ON" class="Bool (strict)"("Val(Sgnl)"="Red Laser ON/OFF") -> ()  [unwired: 2 in, 2 out]
        n1434 = property on="Blue Laser ON" class="Bool (strict)"("Val(Sgnl)"="Blue Laser ON/OFF") -> ()  [unwired: 2 in, 2 out]
        n1435 = property on="Green Laser ON" class="Bool (strict)"("Val(Sgnl)"="Green Laser ON/OFF") -> ()  [unwired: 2 in, 2 out]
      }
      event "Laser interlacing mode", "Green Laser ON", "Red Laser ON", "Blue Laser ON": Value Change {
        n1436 = event-data() -> ()  [unwired: 7 out]
        n1437 = local write "Green Laser ON/OFF"("Green Laser ON") -> ()
        n1438 = local write "Blue Laser ON/OFF"("Blue Laser ON") -> ()
        n1439 = local write "Red Laser ON/OFF"("Red Laser ON") -> ()
        n1440 = case shown="True" "Green Laser ON" {
          tunnel: "Laser interlacing mode" -> [_ w2078]
          tunnel: [enum32{"Laser ON", "Laser OFF", "Interlace"}."Laser OFF" ("Green laser mode") w2078] -> w2054
          tunnel: [FALSE w2074] -> w2053
          frame False {
          }
          frame True {
            n1441 = local read "Green FB On/Off"() -> (w2075:bool)
            n1442 = Equal?(x=w2078, y=enum32{"Laser ON", "Laser OFF", "Interlace"}."Interlace") -> (x = y?=w2076:bool)
            n1443 = And(x=w2076, y=w2075) -> (x .and. y?=w2074:bool)
          }
        }
        n1444 = case shown="True" "Red Laser ON" {
          tunnel: "Laser interlacing mode" -> [_ w2071]
          tunnel: [enum32{"Laser ON", "Laser OFF", "Interlace"}."Laser OFF" ("Green laser mode") w2071] -> w2050
          tunnel: [FALSE w2067] -> w2049
          frame False {
          }
          frame True {
            n1445 = local read "Red FB On/Off"() -> (w2068:bool)
            n1446 = Equal?(x=w2071, y=enum32{"Laser ON", "Laser OFF", "Interlace"}."Interlace") -> (x = y?=w2069:bool)
            n1447 = And(x=w2069, y=w2068) -> (x .and. y?=w2067:bool)
          }
        }
        n1448 = case shown="True" "Blue Laser ON" {
          tunnel: "Laser interlacing mode" -> [_ w2062]
          tunnel: [enum32{"Laser ON", "Laser OFF", "Interlace"}."Laser OFF" ("Green laser mode") w2062] -> w2046
          tunnel: [FALSE w2060] -> w2045
          frame False {
          }
          frame True {
            n1449 = local read "Blue FB On/Off"() -> (w2061:bool)
            n1450 = Equal?(x=w2062, y=enum32{"Laser ON", "Laser OFF", "Interlace"}."Interlace") -> (x = y?=w2063:bool)
            n1451 = And(x=w2063, y=w2061) -> (x .and. y?=w2060:bool)
          }
        }
        n1452 = xnode "Read/Write Control"("FPGA VI Reference In"=w2057, "error in"=w2055, "Operating Mode"=w2054, "Operating Mode 2"=w2054, "Green FB On/Off"=w2053, "Red Laser Operating Mode"=w2050, "RI Operating Mode 2"=w2050, "Red FB On/Off"=w2049, "BI Operating Mode (AO)"=w2046, "Blue Laser Operating Mode (D)"=w2046, "Blue FB On/Off"=w2045) -> ("error out"=w2056:errorcluster)  [unwired: 1 out]
      }
      event "Invert laser interlacing": Value Change {
        n1453 = event-data() -> ()  [unwired: 7 out]
        n1454 = xnode "Read/Write Control"("FPGA VI Reference In"=w2082, "error in"=w2080, "Invert GI"="Invert laser interlacing", "Invert GI 2"="Invert laser interlacing", "Invert RI"="Invert laser interlacing", "Invert RI 2"="Invert laser interlacing", "Invert BI (AO)"="Invert laser interlacing", "Invert BI (D)"="Invert laser interlacing") -> ("error out"=w2081:errorcluster)  [unwired: 1 out]
      }
      event "Green FB Setpoint (mV)", "Green FB Gains", "Green FB On/Off", "Green Intensity % (FB OFF)", "Green int current ON count adj": Value Change {
        n1455 = event-data() -> ()  [unwired: 7 out]
        n1456 = local read "Green FB Setpoint (mV)"() -> (w2093:dbl)
        n1457 = Multiply(x=w2093, y=3.2767) -> (x*y=w2092:dbl)
        n1458 = local read "Green Intensity % (FB OFF)"() -> (w2096:dbl)
        n1459 = Multiply(x=w2096, y=655.35) -> (x*y=w2097:dbl)
        n1460 = To Unsigned Word Integer(number=w2097) -> (unsigned 16bit integer=w2095:u16)
        n1461 = local read "Green int current ON count adj"() -> (w2099:u32)
        n1462 = local read "Laser interlacing mode"() -> (w2089:enum32{"Laser ON", "Laser OFF", "Interlace"})
        n1463 = local read "Green FB Gains"() -> (w2086:T9)
        n1464 = local read "Green Laser ON"() -> (w2090:bool)
        n1465 = local read "Green FB On/Off"() -> (w2100:bool)
        n1466 = Equal?(x=w2089, y=enum32{"Laser ON", "Laser OFF", "Interlace"}."Interlace") -> (x = y?=w2087:bool)
        n1467 = Unbundle By Name(w2086) -> ("proportional gain (Kc)"=w2085:i16, "integral gain (Kc*Ts/Ti)"=w2084:i16, "derivative gain (Kc*Td/Ts)"=w2083:i16)
        n1468 = Compound Arithmetic op=AND(w2087, w2100, w2090) -> (w2091:bool)
        n1469 = xnode "Read/Write Control"("FPGA VI Reference In"=w2103, "error in"=w2102, "Green FB Setpoint"=w2092, "Green FB On/Off"=w2091, "Current Out"=w2095, "Green int current ON count adj"=w2099, "P3"=w2085, "I3"=w2084, "D3"=w2083) -> ("error out"=w2101:errorcluster)  [unwired: 1 out]
      }
      event "Blue FB Setpoint (mV)", "Blue FB Gains", "Blue FB On/Off", "Blue Intensity % (FB OFF)", "Blue int AO ON count adjust": Value Change {
        # "16 bit analog out"
        n1470 = event-data() -> ()  [unwired: 7 out]
        n1471 = Multiply(x="Blue FB Setpoint (mV)", y=3.2767) -> (x*y=w2117:dbl)
        n1472 = Multiply(x="Blue Intensity % (FB OFF)", y=655.35) -> (x*y=w2120:dbl)
        n1473 = To Unsigned Word Integer(number=w2120) -> (unsigned 16bit integer=w2119:u16)
        n1474 = local read "Laser interlacing mode"() -> (w2115:enum32{"Laser ON", "Laser OFF", "Interlace"})
        n1475 = Unbundle By Name("Blue FB Gains") -> ("proportional gain (Kc)"=w2112:i16, "integral gain (Kc*Ts/Ti)"=w2111:i16, "derivative gain (Kc*Td/Ts)"=w2110:i16)
        n1476 = local read "Blue Laser ON"() -> (w2104:bool)
        n1477 = Equal?(x=w2115, y=enum32{"Laser ON", "Laser OFF", "Interlace"}."Interlace") -> (x = y?=w2113:bool)
        n1478 = Compound Arithmetic op=AND(w2113, "Blue FB On/Off", w2104) -> (w2116:bool)
        n1479 = xnode "Read/Write Control"("FPGA VI Reference In"=w2124, "error in"=w2123, "Blue FB Setpoint"=w2117, "Blue FB On/Off"=w2116, "BI Current Out"=w2119, "Blue current ON count adj (AO)"="Blue int AO ON count adjust", "P5"=w2112, "I5"=w2111, "D5"=w2110) -> ("error out"=w2122:errorcluster)  [unwired: 1 out]
      }
      event "Red FB Setpoint (mV)", "Red FB Gains", "Red FB On/Off", "Red Intensity % (FB OFF)": Value Change {
        n1480 = event-data() -> ()  [unwired: 7 out]
        n1481 = local read "Red FB Setpoint (mV)"() -> (w2136:dbl)
        n1482 = Multiply(x=w2136, y=3.2767) -> (x*y=w2135:dbl)
        n1483 = local read "Red Intensity % (FB OFF)"() -> (w2125:dbl)
        n1484 = Multiply(x=w2125, y=655.35) -> (x*y=w2139:dbl)
        n1485 = To Unsigned Word Integer(number=w2139) -> (unsigned 16bit integer=w2138:u16)
        n1486 = local read "Laser interlacing mode"() -> (w2132:enum32{"Laser ON", "Laser OFF", "Interlace"})
        n1487 = local read "Red FB Gains"() -> (w2129:T9)
        n1488 = local read "Red Laser ON"() -> (w2133:bool)
        n1489 = local read "Red FB On/Off"() -> (w2141:bool)
        n1490 = Equal?(x=w2132, y=enum32{"Laser ON", "Laser OFF", "Interlace"}."Interlace") -> (x = y?=w2130:bool)
        n1491 = Unbundle By Name(w2129) -> ("proportional gain (Kc)"=w2128:i16, "integral gain (Kc*Ts/Ti)"=w2127:i16, "derivative gain (Kc*Td/Ts)"=w2126:i16)
        n1492 = Compound Arithmetic op=AND(w2130, w2141, w2133) -> (w2134:bool)
        n1493 = xnode "Read/Write Control"("FPGA VI Reference In"=w2144, "error in"=w2143, "Red FB Setpoint"=w2135, "Red FB On/Off"=w2134, "RI Current Out"=w2138, "P4"=w2128, "I4"=w2127, "D4"=w2126) -> ("error out"=w2142:errorcluster)  [unwired: 1 out]
      }
      event "+ phase (APD 1 Gate)", "- phase (APD 1 Gate)", "+ phase (APD 2 Gate)", "- phase (APD 2 Gate)", "+ phase (APD 3 Gate)", "- phase (APD 3 Gate)", "+ phase (APD Acq)", "- phase (APD Acq)": Value Change {
        n1494 = event-data() -> ()  [unwired: 7 out]
        n1495 = local read "Phase Adj. (APD 1 Gate)"() -> (w2164:i16)
        n1496 = Or(x="- phase (APD 1 Gate)", y="+ phase (APD 1 Gate)") -> (x .or. y?=w2166:bool)
        n1497 = Negate(x=w2164) -> (-x=w2171:i16)
        n1498 = Select(t=w2171, s="+ phase (APD 1 Gate)", f=w2164) -> (s? t:f=w2170:i16)
        n1499 = local read "Phase Adj. (APD 2 Gate)"() -> (w2161:i16)
        n1500 = Or(x="- phase (APD 2 Gate)", y="+ phase (APD 2 Gate)") -> (x .or. y?=w2159:bool)
        n1501 = Negate(x=w2161) -> (-x=w2163:i16)
        n1502 = Select(t=w2163, s="+ phase (APD 2 Gate)", f=w2161) -> (s? t:f=w2160:i16)
        n1503 = Negate(x="Phase Adj. (APD 3 Gate)") -> (-x=w2158:i16)
        n1504 = Or(x="- phase (APD 3 Gate)", y="+ phase (APD 3 Gate)") -> (x .or. y?=w2154:bool)
        n1505 = Select(t=w2158, s="+ phase (APD 3 Gate)", f="Phase Adj. (APD 3 Gate)") -> (s? t:f=w2155:i16)
        n1506 = local read "Phase Adj. (APD Acq)"() -> (w2152:i16)
        n1507 = Or(x="- phase (APD Acq)", y="+ phase (APD Acq)") -> (x .or. y?=w2150:bool)
        n1508 = Negate(x=w2152) -> (-x=w2153:i16)
        n1509 = Select(t=w2153, s="+ phase (APD Acq)", f=w2152) -> (s? t:f=w2151:i16)
        n1510 = xnode "Read/Write Control"("FPGA VI Reference In"=w2173, "error in"=w2172, "Phase count adjustment (APD 1 Gate)"=w2170, "Phase count adjustment (APD 2 Gate)"=w2160, "Phase count adjustment (APD 3 Gate)"=w2155, "Phase Count Adjustment (APD Acq)"=w2151) -> ("FPGA VI Reference Out"=w2168:T20, "error out"=w2169:errorcluster)
        n1511 = xnode "Read/Write Control"("FPGA VI Reference In"=w2168, "error in"=w2169, "+ phase (APD 1 Gate)"=w2166, "+ phase (APD 2 Gate)"=w2159, "+ phase (APD 3 Gate)"=w2154, "+ phase (APD Acq)"=w2150) -> ("error out"=w2167:errorcluster)  [unwired: 1 out]
      }
      event "Invert APD Gate", "APD Gate ON Count", "APD Gate OFF Count", "APD Gate", "APD Integration Time (s)", "APD AO Scale Factor", "Duty Frequency (ON 1/N cycles)", "Interlace ON count", "Interlace OFF count": Value Change {
        n1512 = event-data() -> ()  [unwired: 7 out]
        n1513 = Add(x="Interlace ON count", y="Interlace OFF count") -> (x+y=w2179:u16)
        n1514 = Add(x="APD Gate ON Count", y="APD Gate OFF Count") -> (x+y=w2190:u16)
        n1515 = Multiply(x="Duty Frequency (ON 1/N cycles)", y=w2179) -> (x*y=w2175:u16)
        "Green AI Count" <- w2175
        "Red AI Count" <- w2175
        "Blue AI Count" <- w2175
        n1516 = Subtract(x=w2175, y="Interlace ON count") -> (x-y=w2178:u16)
        n1517 = Multiply(x=w2190, y="Duty Frequency (ON 1/N cycles)") -> (x*y=w2189:u16)
        n1518 = Subtract(x=w2189, y="APD Gate ON Count") -> (x-y=w2188:u16)
        n1519 = local read "DMA Update Period (s)"() -> (w2191:dbl)
        n1520 = Multiply(x="APD Integration Time (s)", y=40000000.0) -> (x*y=w2195:dbl)
        n1521 = Reciprocal(x="APD Integration Time (s)") -> (1/x=→"APD Acq Rate (Hz)":dbl)
        n1522 = To Unsigned Long Integer(number=w2195) -> (unsigned 32bit integer=w2181:u32)
        "APD Int. Count" <- w2181
        n1523 = local read "Number of APDs"() -> (w2174:u8)
        n1524 = Divide(x=w2191, y="APD Integration Time (s)") -> (x/y=w2193:dbl)
        n1525 = Multiply(x=w2174, y=w2193) -> (x*y=w2192:dbl)
        n1526 = local write "APD Samples/FIFO Acq."(w2193) -> ()
        n1527 = local write "APD Elements/DMA read"(w2192) -> ()
        n1528 = xnode "Read/Write Control"("FPGA VI Reference In"=w2199, "error in"=w2198, "Invert APD Gate"="Invert APD Gate", "APD Gate ON Count"="APD Gate ON Count", "APD Gate OFF Count"=w2188, "APD Acq Rate Count"=w2181, "APD Gate Operating Mode"="APD Gate", "APD AO scale factor"="APD AO Scale Factor", "Green interlace ON count"="Interlace ON count", "Green interlace OFF count"=w2178, "Green interlace ON count 2"="Interlace ON count", "Green interlace OFF count 2"=w2178, "Green FB Count"=w2175, "Red interlace ON count"="Interlace ON count", "Red interlace OFF count"="Interlace OFF count", "Blue ON count (AO)"="Interlace ON count", "Blue OFF count (AO)"="Interlace OFF count", "Blue interlace OFF count (D)"="Interlace OFF count", "Blue interlace ON count (D)"="Interlace ON count") -> ("error out"=w2197:errorcluster)  [unwired: 1 out]
      }
      event "Neg. TTrig FPGA": Value Change {
        n1529 = event-data() -> ()  [unwired: 7 out]
        n1530 = xnode "Read/Write Control"("FPGA VI Reference In"=w2202, "error in"=w2201, "TTrig Negate Pos"="Neg. TTrig FPGA") -> ()  [unwired: 2 out]
      }
      event "Test ttrig": Value Change {
        n1531 = event-data() -> ()  [unwired: 7 out]
        n1532 = xnode "Read/Write Control"("FPGA VI Reference In"=w2206, "error in"=w2205, "TTrig?"=TRUE) -> ("error out"=w2204:errorcluster)  [unwired: 1 out]
      }
      event "Number of F/B Scans (AOD)", "Scan Speed (nm/s)", "Scan BD", "Initial delta (MHz)", "Step Size (nm)", "Scan Range (nm)": Value Change {
        w2269 = 123.0  # AOM cal (nm/MHz)
        n1533 = event-data() -> ()  [unwired: 7 out]
        n1534 = local read "BD 1 Frequency 1 (MHz)"() -> (w2252:dbl)
        n1535 = local read "AOM X Cal (nm/MHz)"() -> (w2244:dbl)
        n1536 = local read "X RF Frequency Limits (MHz)"() -> (w2256:T16)
        n1537 = local read "Y RF Frequency Limits (MHz)"() -> (w2253:T16)
        n1538 = local read "BD 2 Frequency 1 (MHz)"() -> (w2258:dbl)
        n1539 = Negate(x="Scan Range (nm)") -> (-x=w2222:dbl)
        n1540 = Divide(x=w2222, y=w2244) -> (x/y=w2226:dbl)
        n1541 = Select(t=w2256, s="Scan BD", f=w2253) -> (s? t:f=w2255:T16)
        n1542 = Select(t=w2252, s="Scan BD", f=w2258) -> (s? t:f=w2257:dbl)
        n1543 = Unbundle By Name(w2255) -> ("Maximum"=w2264:dbl, "Minimum"=w2263:dbl)
        n1544 = Add(x=w2226, y=w2257) -> (x+y=w2261:dbl)
        n1545 = Divide(x=w2222, y="Step Size (nm)") -> (x/y=w2241:dbl)
        n1546 = Divide(x="Step Size (nm)", y=w2244) -> (x/y=w2250:dbl)
        n1547 = Absolute Value(x=w2241) -> (abs(x)=w2225:dbl)
        n1548 = Sign(1:w2222) -> (0:w2223:dbl)
        n1549 = In Range and Coerce(upper limit=w2264, x=w2261, lower limit=w2263) -> (coerced(x)=w2260:dbl, In Range?=w2262:bool)
        n1550 = To Unsigned Quad Integer(1:w2225) -> (0:w2240:u64)
        "Scan steps (AOD)" <- w2240
        n1551 = call "IR AOM freq to word.vi"("Frequency In (MHz)"=w2250) -> ("Frequency Word Out (double)"=w2247:dbl)
        n1552 = Multiply(x=w2223, y=w2247) -> (x*y=w2224:dbl)
        n1553 = Subtract(x=w2261, y=w2260) -> (x-y=w2259:dbl)
        n1554 = To Quad Integer(1:w2224) -> (0:w2246:i64)
        "Incr. int (AOD)" <- w2246
        n1555 = Subtract(x=w2226, y=w2259) -> (x-y=w2245:dbl)
        "Scan Range (MHz)" <- w2245
        n1556 = Select(t=w2226, s=w2262, f=w2245) -> (s? t:f=w2265:dbl)
        n1557 = Multiply(x=w2245, y=w2244) -> (x*y=w2243:dbl)
        n1558 = Decrement(x=w2240) -> (x-1=w2293:u64)
        n1559 = Negate(x=w2243) -> (-x=w2239:dbl)
        n1560 = local write "Scan Range (nm)"(w2239) -> ()
        n1561 = Divide(x=w2265, y=w2293) -> (x/y=w2249:dbl)
        "Scan Increment (MHz)" <- w2249
        n1562 = call "IR AOM freq to word.vi"("Frequency In (MHz)"=w2249) -> ("Frequency Word Out (double)"=w2248:dbl)
        n1563 = Divide(x="Step Size (nm)", y="Scan Speed (nm/s)") -> (x/y=w2236:dbl)
        n1564 = To Quad Integer(1:w2248) -> ()  [unwired: 1 out]
        n1565 = local read "Number Interlace Sets"() -> (w2220:u8)
        n1566 = local read "AI Count (ticks)"() -> (w2221:u16)
        n1567 = local read "Total Counts (ticks)"() -> (w2219:u16)
        n1568 = local read "# Samples/trap"() -> (w2251:u32)
        n1569 = Multiply(x=w2221, y=w2220) -> (x*y=w2218:u16)
        n1570 = Divide(x=w2219, y=w2218) -> (x/y=w2217:dbl)
        n1571 = Select(t=w2252, s="Scan BD", f=w2258) -> (s? t:f=w2290:dbl)
        "Initial freq. (MHz)" <- w2290
        n1572 = Add(x=w2265, y=w2290) -> (x+y=→"Final freq. (MHz)":dbl)
        n1573 = Divide(x=w2219, y=40000000.0) -> (x/y=w2235:dbl)
        n1574 = Divide(x=w2236, y=w2235) -> (x/y=w2234:dbl)
        n1575 = To Unsigned Quad Integer(1:w2234) -> (0:w2209:u64)
        n1576 = Quotient & Remainder(x=w2209, y=u64 2) -> (x-y*floor(x/y)=w2213:u64)  [unwired: 1 out]
        n1577 = Equal?(x=w2213, y=u64 0) -> (x = y?=w2211:bool)